vi "UHR-Fleezers Control (host) - 10.8MV_trial2.vi"() -> ()   [LabVIEW 2010] (continued)
      tunnel: w5479 -> [w6483 w6488]
      tunnel: [w6483 w6485] -> w5476
      frame False {
      }
      frame True {
        n1529 = Subtract(x=w6490, y=w6486) -> (x-y=w6487:dbl)
        n1530 = Array Subset(array=w6491, index=w6487, length=w6486) -> (w6489:u32[])
        n1531 = Array Subset(array=w6488, index=w6487, length=w6486) -> (w6485:u32[])
      }
    }
    n1532 = feedback-in #3(w5541) -> ()
    n1533 = feedback-in #4(w5476) -> ()
    n1534 = Or(x=w5611, y=w5607) -> (x .or. y?=w5608:bool)
    n1535 = Square Root(x=w5391) -> (sqrt(x)=w5390:dbl)
    n1536 = Equal?(x="Tab Control 6", y=T37."High Res Display") -> (x = y?=w5531:bool)
    n1537 = Multiply(x="APD Disp. Scale", y=w5481) -> (x*y=w5490:waveform(dbl)[])
    n1538 = Multiply(x="APD Disp. Downsample", y=w5488) -> (x*y=w5486:dbl)
    n1539 = Multiply(x=10.0, y=w5390) -> (x*y=→"Trap 1 Position RMS (A)":dbl)
    n1540 = Divide(x=w5490, y=w5486) -> (x/y=w5458:waveform(dbl)[])
    n1541 = Index Array(array=w5458, index=0) -> (element=w5468:waveform(dbl))
    n1542 = case "For computing FFTs for display" shown="True" "Compute FFT" {
      tunnel: w5485 -> [_ w7811]
      frame False {
      }
      frame True {
        n1543 = Build Array("FFT 1 Choice 1", "FFT 1 Choice 2", "FFT 2 Choice 1", "FFT 2 Choice 2") -> (w7804:u16[])
        n1544 = Array Size(array=w7811) -> (size(s)=w7810:i32)
        n1545 = feedback-in #6(w7804) -> ()
        n1546 = feedback #6(u16[] [100, 100, 100, 100]) -> (w7805:u16[])
        n1547 = feedback-in #7("# Spectra to Ave.") -> ()
        n1548 = feedback #7("# Spectra to Ave.") -> (w7802:dbl)
        n1549 = Not Equal?(x="# Spectra to Ave.", y=w7802) -> (x != y?=w7801:bool)
        n1550 = Not Equal?(x=w7804, y=w7805) -> (x != y?=w7803:bool)
        n1551 = feedback #8(1.0) -> (w7788:dbl)
        n1552 = Compound Arithmetic op=OR("Reset FFT", w7803, w7801) -> (w7786:bool)
        n1553 = Select(t=1.0, s=w7786, f=w7788) -> (s? t:f=w7790:dbl)
        n1554 = Greater?(x=w7790, y="# Spectra to Ave.") -> (0:w7809:bool)
        n1555 = Increment(x=w7790) -> (x+1=w7789:dbl)
        n1556 = feedback-in #8(w7789) -> ()
        n1557 = local read "DMA Update Period (s)"() -> (w7784:dbl)
        n1558 = Multiply(x="# Spectra to Ave.", y=w7784) -> (x*y=→"Ave. Time (s)":dbl)
        n1559 = Build Array(cluster{"f0":dbl, "df":dbl, "magnitude":dbl[]} {"f0"=0.0, "df"=0.0, "magnitude"=[]} ("PSD")) -> (w7793:cluster{"f0":dbl, "df":dbl, "magnitude":dbl[]}[])
        n1560 = Build Array(w7793, w7793, w7793, w7793) -> (w7795:T49)
        n1561 = feedback #9(w7795) -> (w7800:T49)
        n1562 = for {
          N: 4 -> [_]
          tunnel: w7804 -> [w7833] mode=indexing
          tunnel: w7811 -> [w7834]
          tunnel: w7810 -> [w7836]
          tunnel: w7786 -> [w7829]
          tunnel: w7809 -> [w7828]
          tunnel: "# Spectra to Ave." -> [w7827]
          tunnel: [w7826] -> w7799 mode=indexing
          tunnel: w7800 -> [w7831] mode=indexing
          tunnel: [w7830] -> w7787 mode=indexing
          tunnel: w7790 -> [w7825]
          n1563 = Less?(x=w7833, y=w7836) -> (x < y?=w7835:bool)
          n1564 = Index Array(array=w7834, index=w7833) -> (element=w7832:waveform(dbl))
          n1565 = case shown="True" w7835 {
            tunnel: w7832 -> [_ w7853]
            tunnel: w7831 -> [w7838 w7851]
            tunnel: [w7838 w7839] -> w7830
            tunnel: w7829 -> [_ w7850]
            tunnel: w7828 -> [_ w7843]
            tunnel: w7827 -> [_ w7842]
            tunnel: [cluster{"f0":dbl, "df":dbl, "magnitude":dbl[]} {"f0"=0.0, "df"=0.0, "magnitude"=[]} ("PSD") w7844] -> w7826
            tunnel: w7825 -> [_ w7841]
            frame False {
            }
            frame True {
              n1566 = call <vilib>:"Std Deviation and Variance.vi"("X"=w7853) -> ("mean"=w7854:dbl)  [unwired: 1 in, 2 out]
              n1567 = Subtract(x=w7853, y=w7854) -> (x-y=w7852:waveform(dbl))
              n1568 = xnode "Spectral Measurements"("Signals"=w7852) -> ("PSD"=w7846:cluster{"f0":dbl, "df":dbl, "magnitude":dbl[]})  [unwired: 1 in, 1 out]
              n1569 = case shown="False" w7850 {
                tunnel: w7851 -> [w7863 _]
                tunnel: [w7859 w7868] -> w7839
                tunnel: w7846 -> [w7862 w7869]
                tunnel: w7843 -> [w7861 _]
                frame False {
                  n1570 = Build Array (concatenate)(w7863, w7862) -> (w7860:cluster{"f0":dbl, "df":dbl, "magnitude":dbl[]}[])
                  n1571 = case shown="True" w7861 {
                    tunnel: w7860 -> [w7864 w7867]
                    tunnel: [w7864 w7865] -> w7859
                    frame False {
                    }
                    frame True {
                      n1572 = Delete From Array(array=w7867, index=0) -> (array with subset deleted=w7865:cluster{"f0":dbl, "df":dbl, "magnitude":dbl[]}[])  [unwired: 1 in, 1 out]
                    }
                  }
                }
                frame True {
                  n1573 = Build Array(w7869) -> (w7868:cluster{"f0":dbl, "df":dbl, "magnitude":dbl[]}[])
                }
              }
              n1574 = for {
                tunnel: w7839 -> [w7858] mode=indexing
                tunnel: [w7857] -> w7849 mode=indexing
                workers-P: _ -> [_]
                n1575 = Unbundle By Name(w7858) -> ("magnitude"=w7857:dbl[])
              }
              n1576 = Transpose 2D Array(2D array=w7849) -> (transposed array=w7848:dbl[][])
              n1577 = for {
                tunnel: w7848 -> [w7856] mode=indexing
                tunnel: [w7855] -> w7847 mode=indexing
                workers-P: _ -> [_]
                n1578 = Add Array Elements(numeric array=w7856) -> (sum=w7855:dbl)
              }
              n1579 = Select(t=w7842, s=w7843, f=w7841) -> (s? t:f=w7840:dbl)
              n1580 = Divide(x=w7847, y=w7840) -> (x/y=w7845:dbl[])
              n1581 = Bundle By Name(cluster=w7846, "magnitude"=w7845) -> (w7844:cluster{"f0":dbl, "df":dbl, "magnitude":dbl[]})
            }
          }
        }
        n1582 = case shown="True" w7786 {
          tunnel: w7787 -> [w7818 w7824]
          tunnel: [w7818 w7819] -> w7785
          frame False {
          }
          frame True {
            n1583 = Array Subset(array=w7824, index (row)=0 ("index"), length (row)=4 ("length"), index (col)=0 ("index"), length (col)=1 ("length")) -> (w7819:T49)
          }
        }
        n1584 = feedback-in #9(w7785) -> ()
        n1585 = Split 1D Array(array=w7799, index=2) -> (first subarray=→"FFT 1":cluster{"f0":dbl, "df":dbl, "magnitude":dbl[]}[], second subarray=→"FFT 2":cluster{"f0":dbl, "df":dbl, "magnitude":dbl[]}[])
      }
    }
    n1586 = Index Array(array=w5458, index=1) -> (element=w5466:waveform(dbl))
    n1587 = case "For displaying the high resolution display (no downsampling)" shown="True" w5531 {
      tunnel: w5485 -> [_ w5993]
      frame False {
      }
      frame True {
        n1588 = Index Array(array=w5993, index="High Res. Display") -> (element=w5994:waveform(dbl))
        n1589 = call <vilib>:"Std Deviation and Variance.vi"("X"=w5994) -> ("mean"=w6001:dbl, "standard deviation"=w6006:dbl)  [unwired: 1 in, 1 out]
        "Mean Intensity" <- w6001
        "Sigma" <- w6006
        n1590 = Subtract(x=w5994, y=w6001) -> (x-y=w6000:waveform(dbl))
        n1591 = Select(t=w6000, s="Subtract mean", f=w5994) -> (s? t:f=→"1 Channel":waveform(dbl))
        n1592 = Divide(x=w6006, y=w6001) -> (x/y=→"Sigma/Mean":dbl)
        n1593 = feedback #10(1) -> (w5995:i32)
        n1594 = Greater Or Equal?(x=w5995, y="Slow mean N ave.") -> (x >= y?=w6008:bool)
        n1595 = Increment(x=w5995) -> (x+1=w6010:i32)
        n1596 = Select(t=1, s=w6008, f=w6010) -> (s? t:f=w5997:i32)
        n1597 = feedback-in #10(w5997) -> ()
        n1598 = feedback #11() -> (w5998:waveform(dbl))  [unwired: 1 out]
        n1599 = case shown="Default" w5995 {
          tunnel: [w6013 w6016] -> w5999
          tunnel: w5998 -> [w6015 _]
          tunnel: w5994 -> [w6014 w6016]
          frame Default {
            n1600 = call-poly <vilib>:"Append Waveforms.vi"("waveform B"=w6014, "waveform A"=w6015) -> ("waveform out"=w6013:waveform(dbl))  [unwired: 1 in, 8 out]
          }
          frame 1 {
          }
        }
        n1601 = feedback-in #11(w5999) -> ()
        n1602 = case shown="True" w6008 {
          tunnel: w5999 -> [_ w6012]
          frame False {
          }
          frame True {
            n1603 = call <vilib>:"Mean.vi"("X"=w6012) -> ("mean"=→"Slow mean":dbl)  [unwired: 1 out]
          }
        }
      }
    }
    n1604 = case "For plotting results of scanning MCL" shown="True" w5608 {
      tunnel: w5607 -> [_ w6524]
      tunnel: w5524 -> [_ w6620]
      tunnel: w5616 -> [_ _]
      tunnel: w5485 -> [_ w6594]
      tunnel: w5460 -> [_ w6525]
      tunnel: w5459 -> [_ w6498]
      frame False {
      }
      frame True {
        w6505 = u32 0 items=["Horizontal", "Vertical", "Central", "1st Diagonal", "2nd Diagonal"] ("Type of Symmetry")
        w6533 = u32 0 items=["Horizontal", "Vertical", "Central", "1st Diagonal", "2nd Diagonal"] ("Type of Symmetry")
        w6536 = u32 0 items=["Horizontal", "Vertical", "Central", "1st Diagonal", "2nd Diagonal"] ("Type of Symmetry")
        w6565 = u32 0 items=["Horizontal", "Vertical", "Central", "1st Diagonal", "2nd Diagonal"] ("Type of Symmetry")
        n1605 = Index Array(array=w6594, index=10) -> (element=w6600:waveform(dbl))
        n1606 = Index Array(array=w6594, index=11) -> (element=w6597:waveform(dbl))
        n1607 = local read "Cycles/step (MCL)"() -> (w6550:u64)
        n1608 = Index Array(array=w6594, index="Channel") -> (element=w6596:waveform(dbl))
        n1609 = Unbundle(w6498) -> ("New Image"=w6497:T2, "New Image"=w6496:T2, "New Image"=w6495:T2, "New Image"=w6494:T2)
        n1610 = Unbundle By Name(w6600) -> ("Y"=w6552:dbl[])
        n1611 = Unbundle By Name(w6597) -> ("Y"=w6554:dbl[])
        n1612 = Unbundle By Name(w6596) -> ("Y"=w6559:dbl[])
        n1613 = call "downsample 1D array - double.vi"("Ave N"=w6550, "Array In"=w6552) -> ("Array Out"=w6551:dbl[])  [unwired: 1 out]
        n1614 = call "downsample 1D array - double.vi"("Ave N"=w6550, "Array In"=w6554) -> ("Array Out"=w6553:dbl[])  [unwired: 1 out]
        n1615 = call "downsample 1D array - double.vi"("Ave N"=w6550, "Array In"=w6559) -> ("Array Out"=w6558:dbl[])  [unwired: 1 out]
        n1616 = feedback #12(w6620) -> (w6621:dbl[])
        n1617 = Build Array (concatenate)(w6621, w6620) -> (w6602:dbl[])
        n1618 = feedback #13(w6525) -> (w6527:dbl[])
        n1619 = Build Array (concatenate)(w6527, w6525) -> (w6526:dbl[])
        n1620 = local read "Scan steps (MCL)"() -> (w6507:u64)
        n1621 = Select(t=w6620, s=w6524, f=w6602) -> (s? t:f=w6606:dbl[])
        n1622 = feedback-in #12(w6606) -> ()
        n1623 = Select(t=w6525, s=w6524, f=w6526) -> (s? t:f=w6508:dbl[])
        n1624 = feedback-in #13(w6508) -> ()
        n1625 = local read "Scan lines (y)"() -> (w6493:u64)
        n1626 = local read "N APD Samp/step"() -> (w6509:dbl)
        n1627 = feedback #14(w6551) -> (w6608:dbl[])
        n1628 = Build Array (concatenate)(w6608, w6551) -> (w6599:dbl[])
        n1629 = feedback #15(w6558) -> (w6618:dbl[])
        n1630 = Build Array (concatenate)(w6618, w6558) -> (w6617:dbl[])
        n1631 = feedback #16(w6553) -> (w6610:dbl[])
        n1632 = Build Array (concatenate)(w6610, w6553) -> (w6611:dbl[])
        n1633 = Select(t=w6551, s=w6524, f=w6599) -> (s? t:f=w6555:dbl[])
        n1634 = feedback-in #14(w6555) -> ()
        n1635 = Select(t=w6558, s=w6524, f=w6617) -> (s? t:f=w6557:dbl[])
        n1636 = feedback-in #15(w6557) -> ()
        n1637 = Select(t=w6553, s=w6524, f=w6611) -> (s? t:f=w6556:dbl[])
        n1638 = feedback-in #16(w6556) -> ()
        n1639 = Multiply(x=w6507, y=u64 2) -> (x*y=w6492:u64)
        n1640 = call "integrate 1D array interval - double.vi"("Ave N"=w6509, "Array In"=w6508) -> ("Array Out"=w6520:dbl[])  [unwired: 1 out]
        n1641 = call "integrate 1D array interval - double.vi"("Ave N"=w6509, "Array In"=w6606) -> ("Array Out"=w6605:dbl[])  [unwired: 1 out]
        n1642 = Array Size(array=w6520) -> (size(s)=w6521:i32)
        n1643 = Array Size(array=w6605) -> (size(s)=w6607:i32)
        n1644 = Multiply(x=w6493, y=w6492) -> (x*y=w6523:u64)
        n1645 = Multiply(x=w6493, y=w6492) -> (x*y=w6615:u64)
        n1646 = call <vilib>:"Mean.vi"("X"=w6555) -> ("mean"=w6539:dbl)  [unwired: 1 out]
        n1647 = Subtract(x=w6523, y=w6521) -> (x-y=w6514:u64)
        n1648 = call <vilib>:"Mean.vi"("X"=w6557) -> ("mean"=w6544:dbl)  [unwired: 1 out]
        n1649 = call <vilib>:"Mean.vi"("X"=w6556) -> ("mean"=w6542:dbl)  [unwired: 1 out]
        n1650 = call <vilib>:"Mean.vi"("X"=w6520) -> ("mean"=w6511:dbl)  [unwired: 1 out]
        n1651 = Subtract(x=w6615, y=w6607) -> (x-y=w6549:u64)
        n1652 = call <vilib>:"Mean.vi"("X"=w6605) -> ("mean"=w6546:dbl)  [unwired: 1 out]
        n1653 = Initialize Array(1.0 ("element"), w6514) -> (w6510:dbl[])
        n1654 = Initialize Array(1.0 ("element"), w6549) -> (w6540:dbl[])
        n1655 = Multiply(x=w6510, y=w6511) -> (x*y=w6512:dbl[])
        n1656 = Multiply(x=w6540, y=w6542) -> (x*y=w6543:dbl[])
        n1657 = Multiply(x=w6540, y=w6544) -> (x*y=w6545:dbl[])
        n1658 = Multiply(x=w6540, y=w6539) -> (x*y=w6541:dbl[])
        n1659 = Multiply(x=w6540, y=w6546) -> (x*y=w6547:dbl[])
        n1660 = Build Array (concatenate)(w6555, w6541) -> (w6609:dbl[])
        n1661 = Build Array (concatenate)(w6557, w6545) -> (w6613:dbl[])
        n1662 = Build Array (concatenate)(w6556, w6543) -> (w6612:dbl[])
        n1663 = Build Array (concatenate)(w6520, w6512) -> (w6522:dbl[])
        n1664 = Build Array (concatenate)(w6605, w6547) -> (w6614:dbl[])
        n1665 = Reshape Array(w6609, w6493, w6492) -> (w6575:dbl[][])
        n1666 = Reshape Array(w6522, w6493, w6492) -> (w6518:dbl[][])
        n1667 = Reshape Array(w6613, w6493, w6492) -> (w6567:dbl[][])
        n1668 = Reshape Array(w6612, w6493, w6492) -> (w6582:dbl[][])
        n1669 = Reshape Array(w6614, w6493, w6492) -> (w6592:dbl[][])
        n1670 = Array Subset(array=w6582, index (col)=0 ("index"), length (col)=w6507) -> (w6587:dbl[][])  [unwired: 2 in]
        n1671 = Array Subset(array=w6582, index (col)=w6507) -> (w6585:dbl[][])  [unwired: 3 in]
        n1672 = Array Subset(array=w6567, index (col)=0 ("index"), length (col)=w6507) -> (w6573:dbl[][])  [unwired: 2 in]
        n1673 = Array Subset(array=w6567, index (col)=w6507) -> (w6571:dbl[][])  [unwired: 3 in]
        n1674 = Array Subset(array=w6518, index (col)=0 ("index"), length (col)=w6507) -> (w6517:dbl[][])  [unwired: 2 in]
        n1675 = Array Subset(array=w6518, index (col)=w6507) -> (w6515:dbl[][])  [unwired: 3 in]
        n1676 = Array Subset(array=w6592, index (col)=0 ("index"), length (col)=w6507) -> (w6591:dbl[][])  [unwired: 2 in]
        n1677 = Array Subset(array=w6592, index (col)=w6507) -> (w6589:dbl[][])  [unwired: 3 in]
        n1678 = Array Subset(array=w6575, index (col)=0 ("index"), length (col)=w6507) -> (w6580:dbl[][])  [unwired: 2 in]
        n1679 = Array Subset(array=w6575, index (col)=w6507) -> (w6578:dbl[][])  [unwired: 3 in]
        n1680 = for {
          tunnel: w6587 -> [w6629] mode=indexing
          tunnel: [w6628] -> w6586 mode=indexing
          workers-P: _ -> [_]
          n1681 = Reverse 1D Array(array=w6629) -> (reversed array=w6628:dbl[])
        }
        n1682 = for {
          tunnel: w6573 -> [w6625] mode=indexing
          tunnel: [w6624] -> w6572 mode=indexing
          workers-P: _ -> [_]
          n1683 = Reverse 1D Array(array=w6625) -> (reversed array=w6624:dbl[])
        }
        n1684 = for {
          tunnel: w6517 -> [w6623] mode=indexing
          tunnel: [w6622] -> w6516 mode=indexing
          workers-P: _ -> [_]
          n1685 = Reverse 1D Array(array=w6623) -> (reversed array=w6622:dbl[])
        }
        n1686 = for {
          tunnel: w6591 -> [w6631] mode=indexing
          tunnel: [w6630] -> w6590 mode=indexing
          workers-P: _ -> [_]
          n1687 = Reverse 1D Array(array=w6631) -> (reversed array=w6630:dbl[])
        }
        n1688 = for {
          tunnel: w6580 -> [w6627] mode=indexing
          tunnel: [w6626] -> w6579 mode=indexing
          workers-P: _ -> [_]
          n1689 = Reverse 1D Array(array=w6627) -> (reversed array=w6626:dbl[])
        }
        n1690 = Index Array(array=w6592, index (row)=0) -> (element=→"Waveform Graph":dbl[])  [unwired: 1 in]
        n1691 = Add(x=w6586, y=w6585) -> (x+y=w6584:dbl[][])
        n1692 = Add(x=w6572, y=w6571) -> (x+y=w6570:dbl[][])
        n1693 = Add(x=w6516, y=w6515) -> (x+y=w6500:dbl[][])
        n1694 = Add(x=w6590, y=w6589) -> (x+y=w6564:dbl[][])
        n1695 = Add(x=w6579, y=w6578) -> (x+y=w6577:dbl[][])
        n1696 = Divide(x=w6570, y=2) -> (x/y=w6568:dbl[][])
        n1697 = Divide(x=w6584, y=2) -> (x/y=w6529:dbl[][])
        n1698 = Divide(x=w6577, y=2) -> (x/y=w6531:dbl[][])
        n1699 = To Single Precision Float(number=w6564) -> (single precision float=w6563:sgl[][])
        n1700 = Transpose 2D Array(2D array=w6568) -> (transposed array=→"Data map":dbl[][])
        n1701 = To Single Precision Float(number=w6500) -> (single precision float=w6504:sgl[][])
        n1702 = To Single Precision Float(number=w6529) -> (single precision float=w6535:sgl[][])
        n1703 = To Single Precision Float(number=w6531) -> (single precision float=w6532:sgl[][])
        n1704 = call "IMAQ ArrayToImage"("Image Pixels (Float)"=w6563, "Image"=w6497) -> ("Image Out"=w6566:T2)  [unwired: 8 in, 1 out]
        n1705 = call "IMAQ ArrayToImage"("Image Pixels (Float)"=w6504, "Image"=w6496) -> ("Image Out"=w6506:T2)  [unwired: 8 in, 1 out]
        n1706 = call "IMAQ ArrayToImage"("Image Pixels (Float)"=w6535, "Image"=w6495) -> ("Image Out"=w6537:T2)  [unwired: 8 in, 1 out]
        n1707 = call "IMAQ ArrayToImage"("Image Pixels (Float)"=w6532, "Image"=w6494) -> ("Image Out"=w6534:T2)  [unwired: 8 in, 1 out]
        n1708 = call "IMAQ Symmetry"("Type of Symmetry"=w6565, "Image Src"=w6566) -> ("Image Dst Out"=w6561:T2)  [unwired: 3 in, 1 out]
        n1709 = call "IMAQ Symmetry"("Type of Symmetry"=w6505, "Image Src"=w6506) -> ("Image Dst Out"=w6502:T2)  [unwired: 3 in, 1 out]
        n1710 = call "IMAQ Symmetry"("Type of Symmetry"=w6536, "Image Src"=w6537) -> ("Image Dst Out"=→"Detection Laser X":T2)  [unwired: 3 in, 1 out]
        n1711 = call "IMAQ Symmetry"("Type of Symmetry"=w6533, "Image Src"=w6534) -> ("Image Dst Out"=→"Detection Laser Y":T2)  [unwired: 3 in, 1 out]
        n1712 = call "IMAQ Set Simple Calibration"("Calibration Axis Info"=T38 {"Origin Pixel"={"X"=0.0, "Y"=0.0}, "Angle Relative to Horizontal (deg)"=0.0, "Axis Reference"=0}, "Grid Descriptor"=T39 {"X Step"=0.3, "Y Step"=0.3, "Unit"=enum."Undefined"}, "Image"=w6561) -> ("Calibrated Image"=→"APD 1":T2)  [unwired: 7 in, 1 out]
        n1713 = call "IMAQ Set Simple Calibration"("Calibration Axis Info"=T38 {"Origin Pixel"={"X"=0.0, "Y"=0.0}, "Angle Relative to Horizontal (deg)"=0.0, "Axis Reference"=0}, "Grid Descriptor"=T39 {"X Step"=0.3, "Y Step"=0.3, "Unit"=enum."Undefined"}, "Image"=w6502) -> ("Calibrated Image"=→"APD 2":T2)  [unwired: 7 in, 1 out]
      }
    }
    n1714 = Subtract(x=w5466, y="APD 2 Offset") -> (x-y=w5463:waveform(dbl))
    n1715 = Subtract(x=w5468, y="APD 1 Offset") -> (x-y=w5464:waveform(dbl))
    n1716 = Index Array(array=w5483, index=3) -> (element=w5552:waveform(dbl))
    n1717 = Index Array(array=w5483, index=6) -> (element=w5549:waveform(dbl))
    n1718 = Build Array(w5464, w5463) -> (→"APD Chart":waveform(dbl)[])
    n1719 = Array Size(array=w5541) -> (size(s)=w5596:i32)
    n1720 = call <vilib>:"Std Deviation and Variance.vi"("X"=w5476) -> ("standard deviation"=w5475:dbl)  [unwired: 1 in, 2 out]
    n1721 = Add Array Elements(numeric array=w5476) -> (sum=w5478:u32)
    n1722 = Add Array Elements(numeric array=w5541) -> (sum=w5606:u32)
    n1723 = call <vilib>:"Std Deviation and Variance.vi"("X"=w5541) -> ("standard deviation"=w5540:dbl)  [unwired: 1 in, 2 out]
    n1724 = Divide(x="T1 offset_x (mV)", y=1000.0) -> (x/y=w5553:dbl)
    n1725 = Divide(x=w5475, y=w5474) -> (x/y=w5471:dbl)
    "Rate sigma (Hz) 2" <- w5471
    n1726 = Multiply(x=w5474, y=w5596) -> (x*y=w5477:dbl)
    "Int. Time (s)" <- w5477
    n1727 = Divide(x=w5478, y=w5477) -> (x/y=w5472:dbl)
    "APD 2 Rate (Hz)" <- w5472
    n1728 = Divide(x=w5606, y=w5477) -> (x/y=w5538:dbl)
    "APD 1 Rate (Hz)" <- w5538
    n1729 = Divide(x=w5540, y=w5474) -> (x/y=w5539:dbl)
    "Rate sigma (Hz)" <- w5539
    n1730 = Divide(x=w5471, y=w5472) -> (x/y=→"Sigma/Mean 2":dbl)
    n1731 = Divide(x=w5539, y=w5538) -> (x/y=→"Sigma/Mean":dbl)
    n1732 = Divide(x="T2 offset_x (mV)", y=1000.0) -> (x/y=w5551:dbl)
    n1733 = case shown="1" "Calibration" {
      tunnel: "T1 alpha_x (nm/V)" -> [_ w6460 w6481]
      tunnel: "T1 kappa_x (pN/nm)" -> [_ _ w6471]
      tunnel: "T2 alpha_x (nm/V)" -> [_ w6459 w6479]
      tunnel: "T2 kappa_x (pN/nm)" -> [_ _ w6472]
      tunnel: w5552 -> [w6442 w6457 w6477]
      tunnel: w5549 -> [w6441 w6455 w6475]
      tunnel: [w6442 w6454 w6474] -> w5582
      tunnel: [w6441 w6453 w6473] -> w5581
      tunnel: ["T1 X (V)" ("Label.Text") "T1 X (nm)" ("Label.Text") "T1 X (pN)" ("Label.Text")] -> w5570
      tunnel: ["T2 X (V)" ("Label.Text") "T2 X (nm)" ("Label.Text") "T2 X (pN)" ("Label.Text")] -> w5569
      tunnel: ["Position (V)" ("Label.Text") "Position (nm)" ("Label.Text") "Force (pN)" ("Label.Text")] -> w5571
      tunnel: w5551 -> [_ w6445 w6464]
      tunnel: w5553 -> [_ w6448 w6466]
      tunnel: ["Mean (V)" ("Label.Text") "Mean (nm)" ("Label.Text") "Mean (pN)" ("Label.Text")] -> w5566
      tunnel: ["Difference (V)" ("Label.Text") "Difference (nm)" ("Label.Text") "Difference (pN)" ("Label.Text")] -> w5491
      frame 0, Default {
      }
      frame 1 {
        # "position"
        n1734 = Unbundle By Name(w6457) -> ("Y"=w6461:dbl[])
        n1735 = Unbundle By Name(w6455) -> ("Y"=w6446:dbl[])
        n1736 = Subtract(x=w6461, y=w6448) -> (x-y=w6449:dbl[])
        n1737 = Subtract(x=w6446, y=w6445) -> (x-y=w6447:dbl[])
        n1738 = Multiply(x=w6447, y=w6459) -> (x*y=w6456:dbl[])
        n1739 = Multiply(x=w6460, y=w6449) -> (x*y=w6458:dbl[])
        n1740 = Bundle By Name(cluster=w6455, "Y"=w6456) -> (w6453:waveform(dbl))
        n1741 = Bundle By Name(cluster=w6457, "Y"=w6458) -> (w6454:waveform(dbl))
      }
      frame 2 {
        # "force"
        n1742 = Unbundle By Name(w6477) -> ("Y"=w6482:dbl[])
        n1743 = Unbundle By Name(w6475) -> ("Y"=w6480:dbl[])
        n1744 = Subtract(x=w6480, y=w6464) -> (x-y=w6465:dbl[])
        n1745 = Subtract(x=w6482, y=w6466) -> (x-y=w6467:dbl[])
        n1746 = Compound Arithmetic op=MULTIPLY(w6465, w6479, w6472) -> (w6476:dbl[])
        n1747 = Compound Arithmetic op=MULTIPLY(w6471, w6481, w6467) -> (w6478:dbl[])
        n1748 = Bundle By Name(cluster=w6475, "Y"=w6476) -> (w6473:waveform(dbl))
        n1749 = Bundle By Name(cluster=w6477, "Y"=w6478) -> (w6474:waveform(dbl))
      }
    }
    n1750 = feedback-in #17("Calibration") -> ()
    n1751 = feedback #17(u16 1 ("Calibration")) -> (w5573:u16)
    n1752 = Not Equal?(x=w5573, y="Calibration") -> (x != y?=w5529:bool)
    n1753 = Unbundle By Name(w5552) -> ("Y"=w5555:dbl[])
    n1754 = Unbundle By Name(w5549) -> ("Y"=w5558:dbl[])
    n1755 = Subtract(x=w5555, y=w5553) -> (x-y=w5556:dbl[])
    n1756 = Subtract(x=w5558, y=w5551) -> (x-y=w5557:dbl[])
    n1757 = disable-structure shown="Enabled" {
      disable-tunnel: [-1.0 ("y") 1.0] -> w5559
      frame Disabled {
      }
      frame Enabled {
      }
    }
    n1758 = Multiply(x=w5557, y="T2 alpha_x (nm/V)") -> (x*y=w5548:dbl[])
    n1759 = Multiply(x="T1 alpha_x (nm/V)", y=w5556) -> (x*y=w5547:dbl[])
    n1760 = Multiply(x=w5581, y=w5559) -> (x*y=w5560:waveform(dbl))
    n1761 = case shown="True" "Read Lateness and Rel Phase" {
      tunnel: w5383 -> [w6017 w6039]
      tunnel: w5382 -> [w6018 w6038]
      tunnel: [w6017 w6037] -> w5544
      tunnel: [w6018 w6036] -> w5543
      frame False {
      }
      frame True {
        n1762 = xnode "Read/Write Control"("FPGA VI Reference In"=w6039, "error in"=w6038) -> ("FPGA VI Reference Out"=w6037:T19, "error out"=w6036:errorcluster, "GI Relative phase"=→"GI relative phase":i16, "Relative phase"=→"Relative phase (AI1)":i16, "AI Late Counter"=→"Late Counter (AI1)":u16, "GI Late Counter"=→"GI Late Counter":u16, "MCL Late Counter"=→"MCL Late Counter":u16, "MCL Relative Phase"=→"Relative Phase (MCL)":i16, "APD Acq Relative Phase"=→"APD Acq Relative Phase":i16, "APD 1 Gate Relative Phase"=→"APD 1 Gate Relative Phase":i16, "APD 2 Gate Relative Phase"=→"APD 2 Gate Relative Phase":i16, "APD Acq Late Counter"=→"APD Acq Late Counter":u16, "APD 1 Gate Late Counter"=→"APD 1 Gate Late Counter":u16, "APD 2 Gate Late Counter"=→"APD 2 Gate Late Counter":u16, "Green FB Relative Phase"=→"Relative phase (Green FB)":i16, "GI Relative phase 2"=→"GI relative phase 2":i16, "GI Late Counter 2"=→"GI Late Counter 2":u16, "Trap Pos FIFO Timeout"=→"Trap Pos FIFO Timeout":u16, "Trap AI FIFO Timeout"=→"Trap AI FIFO Timeout":u16)
      }
    }
    n1763 = Subtract(x=w5548, y=w5547) -> (x-y=w5546:dbl[])
    n1764 = Unbundle By Name(w5581) -> ("Y"=w5516:dbl[])
    n1765 = Unbundle By Name(w5582) -> ("Y"=w5517:dbl[])
    n1766 = Build Array(w5582, w5560) -> (→"Force":waveform(dbl)[])
    n1767 = Subtract(x=w5546, y="Offset (nm)") -> (x-y=w5514:dbl[])
    n1768 = call <vilib>:"Mean.vi"("X"=w5516) -> ("mean"=w5495:dbl)  [unwired: 1 out]
    "T2 X" <- w5495
    n1769 = Absolute Value(x=w5517) -> (abs(x)=w5518:dbl[])
    n1770 = Absolute Value(x=w5516) -> (abs(x)=w5519:dbl[])
    n1771 = call <vilib>:"Mean.vi"("X"=w5517) -> ("mean"=w5496:dbl)  [unwired: 1 out]
    "T1 X" <- w5496
    n1772 = Add(x=w5518, y=w5519) -> (x+y=w5520:dbl[])
    n1773 = Bundle By Name(cluster=w5552, "Y"=w5514) -> (w5482:waveform(dbl))
    "Bead Separation" <- w5482
    n1774 = Divide(x=w5520, y=2.0) -> (x/y=→"Vec Mean of T1 T2":dbl[])
    n1775 = case shown="True" w5529 {
      tunnel: w5571 -> [_ w6435]
      tunnel: w5570 -> [_ w6434]
      tunnel: w5569 -> [_ w6433]
      tunnel: w5566 -> [_ w6432]
      tunnel: w5491 -> [_ w6431]
      frame False {
      }
      frame True {
        n1776 = property on="Force" class="WFChart (strict)"("YScale.NameLbl.Text"=w6435) -> ()  [unwired: 2 in, 2 out]
        n1777 = property on="T2 X" class="DigNum (strict)"("Caption.Text"=w6433) -> ()  [unwired: 2 in, 2 out]
        n1778 = property on="T1 X" class="DigNum (strict)"("Caption.Text"=w6434) -> ()  [unwired: 2 in, 2 out]
        n1779 = property on="Mean" class="DigNum (strict)"("Caption.Text"=w6432) -> ()  [unwired: 2 in, 2 out]
        n1780 = property on="Difference" class="DigNum (strict)"("Caption.Text"=w6431) -> ()  [unwired: 2 in, 2 out]
      }
    }
    n1781 = local read "Tether"() -> (w5523:bool)
    n1782 = Absolute Value(x=w5496) -> (abs(x)=w5493:dbl)
    n1783 = Absolute Value(x=w5495) -> (abs(x)=w5492:dbl)
    n1784 = Add(x=w5493, y=w5492) -> (x+y=w5568:dbl)
    n1785 = Subtract(x=w5493, y=w5492) -> (x-y=→"Difference":dbl)
    n1786 = feedback #18(w5514) -> (w5513:dbl[])
    n1787 = Divide(x=w5568, y=2.0) -> (x/y=w5522:dbl)
    "Mean" <- w5522
    n1788 = case shown="True" w5523 {
      tunnel: w5522 -> [_ w5976]
      frame False {
      }
      frame True {
        n1789 = Greater?(x="Lost Tether Alarm Threshold (pN)", y=w5976) -> (0:w5974:bool)
        n1790 = case shown="True" w5974 {
          frame False {
          }
          frame True {
            n1791 = flat-sequence {
              frame #0 {
                # "stop only if saving"
                n1792 = local read "Saving..."() -> (w5989:bool)
                n1793 = And(x=w5989, y="TA Cancel Save?") -> (x .and. y?=w5988:bool)
                n1794 = local write "Stop Saving"(w5988) -> ()
              }
              frame #1 {
                n1795 = case shown="True" "TA Green Off?" {
                  frame False {
                  }
                  frame True {
                    w5992 = FALSE ("Fl. Triggered...")
                    n1796 = local write "Fl. Triggered..."(w5992) -> ()
                    n1797 = property on="Green Laser ON/Interlacing" class="Bool (strict)"("Val(Sgnl)"=w5992) -> ()  [unwired: 2 in, 2 out]
                  }
                }
              }
            }
            n1798 = local read "Time tether formed"() -> (w5983:timestamp)
            n1799 = Get Date/Time In Seconds() -> (seconds since 1Jan1904=w5984:timestamp)
            n1800 = Subtract(x=w5984, y=w5983) -> (x-y=w5982:dbl)
            n1801 = Number To Decimal String(number=w5982) -> (decimal integer string=w5979:string)  [unwired: 1 out]
            n1802 = local read "Messages"() -> (w5986:string)
            n1803 = call <vilib>:"Beep.vi"() -> ()  [unwired: 3 in, 9 out]
            n1804 = Concatenate Strings("Lost tether (" ("Message to add"), w5979, " s)." ("string")) -> (w5981:string)
            n1805 = local write "Tether"(FALSE ("Tether")) -> ()
            n1806 = call "Update messages.vi"("Message to add"=w5981, "Old message string"=w5986) -> ("New message string"=w5985:string)
            n1807 = local write "Messages"(w5985) -> ()
            n1808 = property on="Trap Pos. FB ON" class="Bool (strict)"("Val(Sgnl)"=FALSE ("Value (Signaling)")) -> ()  [unwired: 2 in, 2 out]
          }
        }
      }
    }
    n1809 = Build Array (concatenate)(w5514, w5513) -> (w5512:dbl[])
    n1810 = Split 1D Array(array=w5512, index=w5394) -> (first subarray=w5508:dbl[])  [unwired: 1 out]
    n1811 = feedback-in #18(w5508) -> ()
    n1812 = call <vilib>:"Mean.vi"("X"=w5508) -> ("mean"=w5507:dbl)  [unwired: 1 out]
    "Bead Mean (nm)" <- w5507
    n1813 = Subtract(x=w5508, y=w5507) -> (x-y=w5506:dbl[])
    n1814 = Square(x=w5506) -> (x^2=w5505:dbl[])
    n1815 = call <vilib>:"Mean.vi"("X"=w5505) -> ("mean"=w5504:dbl)  [unwired: 1 out]
    n1816 = Square Root(x=w5504) -> (sqrt(x)=w5503:dbl)
    n1817 = Multiply(x=10.0, y=w5503) -> (x*y=→"RMS (Ang)":dbl)
    n1818 = xnode "Read/Write Control"("FPGA VI Reference In"=w5544, "error in"=w5543) -> ("FPGA VI Reference Out"=w5662:T19, "error out"=w5656:errorcluster, "AI2 Y Sum Set 1"=w5652:i16, "AI2 Y Sum Set 2"=w5651:i16, "AI1 X Set 1"=w5428:fxp<+/-,16,1>, "AI1 X Set 2"=w5427:fxp<+/-,16,1>, "Trap Pos FB Int Signal"=→"Trap Pos FB Int Signal":fxp<+/-,24,9>, "Trap Pos FB Int-Norm Signal"=→"Trap Pos FB Int-Norm Signal":fxp<+/-,16,1>, "Trap Pos FB Action"=w5421:i64, "Scanning"=→"AOD Scanning":bool, "Scan I"=→"AOD Scan I":u64, "Scanning MCL"=w5654:bool, "Scan I (MCL)"=→"MCL Scan I":u64, "Green FB Signals"=w5591:T43)  [unwired: 1 out]
    "MCL Scanning" <- w5654
    "Trap Pos FB Action" <- w5421
    n1819 = local read "AI2 (V)"() -> (w5653:cluster{"Set 1":dbl, "Set 2":dbl})
    n1820 = Bundle By Name(cluster=w5653, "Set 1"=w5652, "Set 2"=w5651) -> (w5649:cluster{"Set 1":dbl, "Set 2":dbl})
    n1821 = Divide(x=w5421, y=327.67) -> (x/y=→"Action (%)":dbl)
    n1822 = local read "Trap X (AI1)"() -> (w5441:T10)
    n1823 = Divide(x=w5649, y=3276.7) -> (x/y=w5648:cluster{"Set 1":dbl, "Set 2":dbl})
    n1824 = local write "AI2 (V)"(w5648) -> ()
    n1825 = Bundle(cluster=w5441, "Trap 1"=w5428, "Trap 2"=w5427) -> (→"Trap X (AI1)":T10)
    n1826 = Divide(x=w5591, y=3276.7) -> (x/y=w5587:T50)
    n1827 = Unbundle By Name(w5587) -> ("Green FB Ch 0"=w5590:dbl, "Green FB Ch 1"=w5589:dbl, "Green FB Ch 2"=w5588:dbl)
    n1828 = Divide(x=w5590, y=w5588) -> (x/y=w5586:dbl)
    n1829 = Divide(x=w5589, y=w5588) -> (x/y=w5585:dbl)
    n1830 = flat-sequence "To save data" {
      tunnel: [w8292] -> w5673
      tunnel: [w8293] -> w5672
      tunnel: w5622 -> [w8286]
      tunnel: w5510 -> [w8290]
      tunnel: ["Save Calibration"] -> w5645
      tunnel: w5642 -> [w8289]
      tunnel: [w8282] -> w5641
      tunnel: [w8279] -> w5640
      tunnel: [w8276] -> w5639
      tunnel: w5621 -> [w8278]
      tunnel: w5527 -> [w8272]
      tunnel: [w8272] -> w5526
      tunnel: ["Start Saving"] -> w5484
      tunnel: [w8266] -> w5410
      tunnel: [w8265] -> w5409
      tunnel: w5673 -> [w8527]
      tunnel: w5672 -> [w8526]
      tunnel: w5411 -> [w8525]
      tunnel: w5645 -> [w8524]
      tunnel: w5641 -> [w8522]
      tunnel: w5640 -> [w8521]
      tunnel: w5639 -> [w8520]
      tunnel: w5497 -> [w8519]
      tunnel: w5536 -> [w8518]
      tunnel: w5526 -> [w8517]
      tunnel: w5484 -> [w8516]
      tunnel: w5482 -> [w8515]
      tunnel: w5458 -> [w8514]
      tunnel: w5410 -> [w8513]
      tunnel: w5409 -> [w8512]
      tunnel: w5408 -> [w8511]
      frame #0 {
        n1831 = Or(x="Save N Sets", y="Start Saving") -> (x .or. y?=w8273:bool)
        n1832 = To Double Precision Float(number=w8289) -> (double precision float=w8283:dbl)
        n1833 = Build Array(w8273, "Save Calibration", w8286, w8278) -> (w8288:bool[])
        n1834 = Compound Arithmetic op=OR("Save Calibration", w8286, w8273, w8278) -> (w8291:bool)
        n1835 = Boolean Array To Number(Boolean array=w8288) -> (number=w8285:u32)
        n1836 = feedback #19(FALSE ("Save APD Data\nwith Trap Data")) -> (w8267:bool)
        n1837 = feedback #20(refnum<k0> refnum) -> (w8294:refnum<file>)
        n1838 = feedback #21(refnum<k0> refnum) -> (w8269:refnum<file>)
        n1839 = feedback #22(FALSE ("Save APD Data\nwith Trap Data")) -> (w8277:bool)
        n1840 = feedback #23(refnum<k0> refnum) -> (w8280:refnum<file>)
        n1841 = feedback #24(0) -> (w8296:i32)
        n1842 = feedback #25() -> (w8284:u32)  [unwired: 1 out]
        n1843 = case shown="True" w8291 {
          tunnel: [w8303 1] -> w8292
          tunnel: w8296 -> [w8305 _]
          tunnel: [w8304 w8323] -> w8293
          tunnel: w8294 -> [w8304 _]
          tunnel: w8290 -> [_ w8343]
          tunnel: w8283 -> [_ w8341]
          tunnel: w8285 -> [_ w8344]
          tunnel: [w8302 w8322] -> w8282
          tunnel: w8284 -> [w8302 _]
          tunnel: [w8301 w8320] -> w8279
          tunnel: w8280 -> [w8301 _]
          tunnel: [w8300 w8319] -> w8276
          tunnel: w8277 -> [w8300 _]
          tunnel: "Start Saving" -> [_ w8317]
          tunnel: w8272 -> [_ w8316]
          tunnel: [w8299 w8307] -> w8265
          tunnel: w8269 -> [w8299 _]
          tunnel: [w8298 w8306] -> w8266
          tunnel: w8267 -> [w8298 _]
          frame False {
            n1844 = Increment(x=w8305) -> (x+1=w8303:i32)
          }
          frame True {
            w8313 = FALSE ("Start Saving")
            w8318 = 9.0  # File Version
            w8326 = FALSE ("prepend array or string size? (T)")
            w8324 = T31."big-endian, network order" ("byte order (0:big-endian, network order)")
            # "write file headers"
            n1845 = local read "BD 1 Frequency 1 (MHz)"() -> (w8340:dbl)
            n1846 = local read "BD 2 Frequency 1 (MHz)"() -> (w8339:dbl)
            n1847 = local read "BD 1 Frequency 2 (MHz)"() -> (w8338:dbl)
            n1848 = local read "BD 2 Frequency 2 (MHz)"() -> (w8337:dbl)
            n1849 = local read "BD 1 Frequency 3 (MHz)"() -> (w8336:dbl)
            n1850 = local read "BD 2 Frequency 3 (MHz)"() -> (w8335:dbl)
            n1851 = Array Size(array=w8316) -> (size(s)=w8315:i32)
            n1852 = To Double Precision Float(number=w8315) -> (double precision float=w8314:dbl)
            n1853 = local write "Save Calibration"(w8313) -> ()
            n1854 = local write "Start Saving"(w8313) -> ()
            n1855 = Build Array("Save APD Data\nwith Trap Data", "Save Trap Pos. Data") -> (w8310:bool[])
            n1856 = Boolean Array To Number(Boolean array=w8310) -> (number=w8309:u32)
            n1857 = Build Array(w8340, w8339, w8338, w8337, w8336, w8335) -> (w8334:dbl[])
            n1858 = case shown="4" w8344 {
              tunnel: w8343 -> [w8415 w8435 w8451 w8489]
              tunnel: w8314 -> [w8420 w8442 w8471 w8508]
              tunnel: w8341 -> [w8419 w8441 w8470 w8507]
              tunnel: [w8416 w8437 w8462 w8499] -> w8332
              tunnel: [w8407 "Cal sets to save" w8452 w8490] -> w8322
              tunnel: w8334 -> [w8417 w8438 w8464 w8501]
              tunnel: "Save APD Data\nwith Trap Data" -> [w8414 _ w8448 w8487]
              tunnel: [w8414 w8429 w8448 w8487] -> w8319
              tunnel: w8318 -> [w8410 w8430 w8446 w8485]
              tunnel: w8317 -> [w8409 _ _ _]
              tunnel: [w8400 w8429 w8445 w8475] -> w8306
              tunnel: "Save Trap Pos. Data" -> [w8400 _ w8445 w8475]
              tunnel: w8309 -> [w8399 _ w8444 w8474]
              frame 1, Default {
                # "timeseries"
                n1859 = case shown="True" "Profile" {
                  tunnel: [w8423 w8426] -> w8404
                  tunnel: [w8423 w8425] -> w8403
                  tunnel: [w8423 w8424] -> w8402
                  tunnel: [w8423 w8428] -> w8401
                  frame False {
                    w8423 = 0.0 ("f")
                  }
                  frame True {
                    n1860 = local read "Current Position"() -> (w8427:dbl[])
                    n1861 = local read "Y change (mm)"() -> (w8428:dbl)
                    n1862 = call "subVI_explode3array.vi"("Array"=w8427) -> ("x"=w8426:dbl, "y"=w8425:dbl, "z"=w8424:dbl)  [unwired: 12 in]
                  }
                }
                n1863 = local read "Save ave N"() -> (w8422:dbl)
                n1864 = Multiply(x=w8422, y=w8415) -> (x*y=w8421:dbl)
                n1865 = To Double Precision Float(number=w8399) -> (double precision float=w8413:dbl)
                n1866 = Build Array(w8410, w8415, w8421, w8420, w8419, 0.0 ("f")) -> (w8418:dbl[])
                n1867 = Build Array(w8413, w8404, w8403, w8402, w8401) -> (w8411:dbl[])
                n1868 = Select(t=u32 4000000000, s=w8409, f="N sets to save") -> (s? t:f=w8407:u32)
                n1869 = Build Array (concatenate)(w8418, w8417, w8411) -> (w8416:dbl[])
              }
              frame 2 {
                w8432 = 0.0 ("f")
                w8429 = FALSE ("Save APD Data\nwith Trap Data")
                # "calibration"
                n1870 = Boolean To (0,1)(Boolean=w8429) -> (0, 1=w8434:i16)
                n1871 = To Double Precision Float(number=w8434) -> (double precision float=w8433:dbl)
                n1872 = Build Array(w8433, w8432, w8432, w8432, w8432) -> (w8431:dbl[])
                n1873 = Build Array(w8430, w8435, w8435, w8442, w8441, 1.0 ("t")) -> (w8439:dbl[])
                n1874 = Build Array (concatenate)(w8439, w8438, w8431) -> (w8437:dbl[])
                "Calibrating Trap..." <- TRUE ("Calibrating...")
              }
              frame 4 {
                w8449 = 0.0 ("f")
                # "write file header for a trap \nraster scan"
                # "scan dir (x/y = 0/1)"
                # "cycles/step"
                # "n scans (f/b)"
                # "steps"
                # "freq. range"
                # "AOD raster scan"
                n1875 = local read "Number of F/B Scans (AOD)"() -> (w8456:u16)
                n1876 = local read "Cycles/step (AOD)"() -> (w8458:u64)
                n1877 = local read "Scan Range (MHz)"() -> (w8461:dbl)
                n1878 = local read "Scan steps (AOD)"() -> (w8460:u64)
                n1879 = local read "Scan BD"() -> (w8468:bool)
                n1880 = local read "Save ave N"() -> (w8473:dbl)
                n1881 = Boolean To (0,1)(Boolean=w8468) -> (0, 1=w8467:i16)
                n1882 = To Double Precision Float(number=w8456) -> (double precision float=w8455:dbl)
                n1883 = To Double Precision Float(number=w8460) -> (double precision float=w8459:dbl)
                n1884 = To Double Precision Float(number=w8458) -> (double precision float=w8457:dbl)
                n1885 = To Double Precision Float(number=w8467) -> (double precision float=w8466:dbl)
                n1886 = Multiply(x=w8473, y=w8451) -> (x*y=w8472:dbl)
                n1887 = To Double Precision Float(number=w8444) -> (double precision float=w8450:dbl)
                n1888 = Build Array(w8450, w8449, w8449, w8449, w8449) -> (w8447:dbl[])
                n1889 = local read "N sets should be saved"() -> (w8453:dbl)
                n1890 = Build Array(w8466, w8461, w8459, w8457, w8455) -> (w8463:dbl[])
                n1891 = Build Array(w8446, w8451, w8472, w8471, w8470, 2.0 ("t")) -> (w8465:dbl[])
                n1892 = Round Toward +Infinity(x=w8453) -> (ceil(x): smallest int >= x=w8454:dbl)
                n1893 = Build Array (concatenate)(w8465, w8464, w8447, w8463) -> (w8462:dbl[])
                n1894 = To Unsigned Long Integer(number=w8454) -> (unsigned 32bit integer=w8452:u32)
              }
              frame 8 {
                w8482 = 0.0 ("f")
                # "MCL raster scan"
                n1895 = local read "Number of scans (MCL)"() -> (w8477:u64)
                n1896 = local read "Scan lines (y)"() -> (w8476:u64)
                n1897 = local read "2D or 1D Scan"() -> (w8479:bool)
                n1898 = local read "Scan Range (V)\n(of steps)"() -> (w8498:dbl)
                n1899 = local read "Fast Scan Dir"() -> (w8505:bool)
                n1900 = local read "Cycles/step (MCL)"() -> (w8495:u64)
                n1901 = local read "Scan steps (MCL)"() -> (w8497:u64)
                n1902 = Select(t=w8476, s=w8479, f=w8477) -> (s? t:f=w8478:u64)
                n1903 = Boolean To (0,1)(Boolean=w8479) -> (0, 1=w8481:i16)
                n1904 = local read "Save ave N"() -> (w8510:dbl)
                n1905 = local read "Initial X"() -> (w8484:dbl)
                n1906 = local read "Initial Y"() -> (w8483:dbl)
                n1907 = To Double Precision Float(number=w8481) -> (double precision float=w8480:dbl)
                n1908 = Boolean To (0,1)(Boolean=w8505) -> (0, 1=w8504:i16)
                n1909 = To Double Precision Float(number=w8478) -> (double precision float=w8493:dbl)
                n1910 = To Double Precision Float(number=w8497) -> (double precision float=w8496:dbl)
                n1911 = To Double Precision Float(number=w8495) -> (double precision float=w8494:dbl)
                n1912 = To Double Precision Float(number=w8504) -> (double precision float=w8503:dbl)
                n1913 = Multiply(x=w8510, y=w8489) -> (x*y=w8509:dbl)
                n1914 = To Double Precision Float(number=w8474) -> (double precision float=w8488:dbl)
                n1915 = local read "N sets should be saved (MCL)"() -> (w8491:dbl)
                n1916 = Build Array(w8488, w8480, w8482, w8482, w8482) -> (w8486:dbl[])
                n1917 = Build Array(w8503, w8498, w8496, w8494, w8493, w8484, w8483) -> (w8500:dbl[])
                n1918 = Build Array(w8485, w8489, w8509, w8508, w8507, 3.0 ("t")) -> (w8502:dbl[])
                n1919 = Round Toward +Infinity(x=w8491) -> (ceil(x): smallest int >= x=w8492:dbl)
                n1920 = Build Array (concatenate)(w8502, w8501, w8486, w8500) -> (w8499:dbl[])
                n1921 = To Unsigned Long Integer(number=w8492) -> (unsigned 32bit integer=w8490:u32)
              }
            }
            n1922 = local read "Index"() -> (w8349:dbl)
            n1923 = call "Create new save file.vi"("Insert"="", "Ext"=".dat", "Index In"=w8349) -> ("Path Out"=w8308:path, "Index Out"=w8321:dbl)
            n1924 = local write "Save file name"(w8308) -> ()
            n1925 = local write "Index"(w8321) -> ()
            n1926 = local write "Save index"(w8321) -> ()
            n1927 = Array Size(array=w8332) -> (size(s)=w8333:i32)
            n1928 = Open/Create/Replace File(file path (use dialog)=w8308, operation (0:open)=T25."create", access (0:read/write)=enum16{"read/write", "read-only", "write-only"}."write-only") -> (refnum out=w8346:refnum<file>)  [unwired: 1 in, 4 out]
            n1929 = local write "Saving..."(TRUE ("Saving...")) -> ()
            n1930 = To Double Precision Float(number=w8333) -> (double precision float=w8331:dbl)
            n1931 = String Length(string="Comment (data description)") -> (length=w8329:i32)
            n1932 = To Double Precision Float(number=w8329) -> (double precision float=w8328:dbl)
            n1933 = Deny Access(7:w8346) -> (3:w8345:refnum<file>)  [unwired: 1 in, 2 out]
            n1934 = Build Array (concatenate)(w8331, w8332, w8328) -> (w8330:dbl[])
            n1935 = case "If fluorescence data to be saved" shown="True" w8319 {
              tunnel: w8308 -> [_ w8398]
              tunnel: [refnum<k0> refnum w8378] -> w8320
              frame False {
              }
              frame True {
                w8377 = 0.0
                n1936 = local read "APD Integration Time (s)"() -> (w8383:dbl)
                n1937 = local read "N APD Samp/step"() -> (w8376:dbl)
                n1938 = Path To String(path=w8398) -> (string=w8397:string)
                n1939 = String Length(string=w8397) -> (length=w8396:i32)
                n1940 = Subtract(x=w8396, y=4) -> (x-y=w8394:i32)
                n1941 = String Subset(string=w8397, length (rest)=w8394) -> (substring=w8393:string)  [unwired: 1 out]
                n1942 = Build Array(w8383, w8376, w8377, w8377, w8377, w8377, w8377, w8377) -> (w8380:dbl[])
                n1943 = Concatenate Strings(w8393, "_fl.dat" ("string")) -> (w8391:string)
                n1944 = Array Size(array=w8380) -> (size(s)=w8382:i32)
                n1945 = String To Path(string=w8391) -> (path=w8387:path)
                n1946 = Open/Create/Replace File(file path (use dialog)=w8387, operation (0:open)=T25."create", access (0:read/write)=enum16{"read/write", "read-only", "write-only"}."write-only") -> (refnum out=w8388:refnum<file>)  [unwired: 1 in, 4 out]
                n1947 = Deny Access(7:w8388) -> (3:w8384:refnum<file>)  [unwired: 1 in, 2 out]
                n1948 = To Double Precision Float(number=w8382) -> (double precision float=w8381:dbl)
                n1949 = Build Array (concatenate)(w8381, w8380) -> (w8379:dbl[])
                n1950 = Write to Binary File(file (use dialog)=w8384, data=w8379, 5:FALSE ("prepend array or string size? (T)"), 9:T31."big-endian, network order" ("byte order (0:big-endian, network order)")) -> (refnum out=w8378:refnum<file>)  [unwired: 1 in, 3 out]
              }
            }
            n1951 = case shown="True" w8306 {
              tunnel: w8308 -> [_ w8360]
              tunnel: [refnum<k0> refnum w8359] -> w8307
              frame False {
              }
              frame True {
                w8355 = 0.0 ("element")
                n1952 = Path To String(path=w8360) -> (string=w8374:string)
                n1953 = Build Array(w8355, w8355, w8355, w8355, w8355, w8355, w8355, w8355) -> (w8356:dbl[])
                n1954 = String Length(string=w8374) -> (length=w8373:i32)
                n1955 = Subtract(x=w8373, y=4) -> (x-y=w8371:i32)
                n1956 = Array Size(array=w8356) -> (size(s)=w8358:i32)
                n1957 = String Subset(string=w8374, length (rest)=w8371) -> (substring=w8370:string)  [unwired: 1 out]
                n1958 = To Double Precision Float(number=w8358) -> (double precision float=w8357:dbl)
                n1959 = Concatenate Strings(w8370, "_pos.dat" ("string")) -> (w8368:string)
                n1960 = Build Array (concatenate)(w8357, w8356) -> (w8354:dbl[])
                n1961 = String To Path(string=w8368) -> (path=w8364:path)
                n1962 = Open/Create/Replace File(file path (use dialog)=w8364, operation (0:open)=T25."create", access (0:read/write)=enum16{"read/write", "read-only", "write-only"}."write-only") -> (refnum out=w8365:refnum<file>)  [unwired: 1 in, 4 out]
                n1963 = Deny Access(7:w8365) -> (3:w8361:refnum<file>)  [unwired: 1 in, 2 out]
                n1964 = Write to Binary File(file (use dialog)=w8361, data=w8354, 5:FALSE ("prepend array or string size? (T)"), 9:T31."big-endian, network order" ("byte order (0:big-endian, network order)")) -> (refnum out=w8359:refnum<file>)  [unwired: 1 in, 3 out]
              }
            }
            n1965 = Write to Binary File(file (use dialog)=w8345, data=w8330, 5:w8326, 9:w8324) -> (refnum out=w8327:refnum<file>)  [unwired: 1 in, 3 out]
            n1966 = Write to Binary File(file (use dialog)=w8327, data="Comment (data description)", 5:w8326, 9:w8324) -> (refnum out=w8323:refnum<file>)  [unwired: 1 in, 3 out]
          }
        }
        n1967 = feedback-in #19(w8266) -> ()
        n1968 = feedback-in #20(w8293) -> ()
        n1969 = feedback-in #21(w8265) -> ()
        n1970 = feedback-in #22(w8276) -> ()
        n1971 = feedback-in #23(w8279) -> ()
        n1972 = feedback-in #24(w8292) -> ()
        n1973 = feedback-in #25(w8282) -> ()
      }
      frame #1 {
        n1974 = local read "Saving..."() -> (w8523:bool)
        n1975 = case shown="True" w8523 {
          tunnel: w8527 -> [_ w8537]
          tunnel: w8526 -> [_ w8551]
          tunnel: w8525 -> [_ w8547]
          tunnel: w8524 -> [_ w8546]
          tunnel: w8522 -> [_ w8545]
          tunnel: w8521 -> [_ w8540]
          tunnel: w8520 -> [_ w8539]
          tunnel: w8519 -> [_ w8538]
          tunnel: w8518 -> [_ w8536]
          tunnel: w8517 -> [_ w8534]
          tunnel: w8516 -> [_ w8533]
          tunnel: w8515 -> [_ w8532]
          tunnel: w8514 -> [_ w8531]
          tunnel: w8513 -> [_ w8530]
          tunnel: w8512 -> [_ w8529]
          tunnel: w8511 -> [_ w8528]
          frame False {
          }
          frame True {
            n1976 = Multiply(x=w8537, y=w8536) -> (x*y=→"Time (s)":dbl)
            n1977 = Less Or Equal?(x=w8537, y=w8545) -> (x <= y?=w8549:bool)
            n1978 = Or(x="Stop Saving", y="Abort save 2") -> (x .or. y?=w8541:bool)
            n1979 = Not(x=w8541) -> (.not. x?=w8550:bool)
            n1980 = And(x=w8549, y=w8550) -> (x .and. y?=w8548:bool)
            n1981 = case shown="False" w8548 {
              tunnel: w8551 -> [w8558 w8626]
              tunnel: [0.0 w8629] -> w8544
              tunnel: w8537 -> [_ w8627]
              tunnel: w8545 -> [_ w8628]
              tunnel: w8547 -> [_ w8623]
              tunnel: w8546 -> [_ _]
              tunnel: w8540 -> [w8556 w8616]
              tunnel: w8539 -> [w8555 w8617]
              tunnel: w8538 -> [_ w8615]